vi "UHR-Fleezers Control (host) - 12.7.vi"() -> ()   [LabVIEW 2012] (continued)
                                }
                                frame #6 {
                                n1115 = property on="Rem fb disp offset" class="Bool (strict)"("Val(Sgnl)"=TRUE ("Value (Signaling)")) -> ()  [unwired: 2 in, 2 out]
                                }
                                }
                                }
                                frame True {
                                n1116 = flat-sequence {
                                tunnel: w1651 -> [w1652]
                                frame #0 {
                                n1117 = property on="Trap Delta (MHz)" class="DigNum (strict)"("Val(Sgnl)"=w1652) -> ()  [unwired: 2 in, 2 out]
                                }
                                frame #1 {
                                n1118 = Wait (ms)(milliseconds to wait=u32 500) -> ()  [unwired: 1 out]
                                }
                                frame #2 {
                                n1119 = local read "Shift confocal"() -> (w1658:bool)
                                n1120 = local read "Mean"() -> (w1660:dbl)
                                n1121 = Greater?(x=w1660, y=11.0) -> (0:w1657:bool)
                                n1122 = Not(x=w1657) -> (.not. x?=w1656:bool)
                                n1123 = And(x=w1657, y=w1658) -> (x .and. y?=w1655:bool)
                                n1124 = And(x=w1656, y=w1658) -> (x .and. y?=w1654:bool)
                                n1125 = case shown="True" w1655 {
                                frame False {
                                }
                                frame True {
                                n1126 = local read "Confocal Y 2 (V)"() -> (w1664:dbl)
                                n1127 = local read "Confocal X 2 (V)"() -> (w1663:dbl)
                                n1128 = property on="AO2" class="Slide (strict)"("Val(Sgnl)"=w1663) -> ()  [unwired: 2 in, 2 out]
                                n1129 = property on="AO1" class="Slide (strict)"("Val(Sgnl)"=w1664) -> ()  [unwired: 2 in, 2 out]
                                }
                                }
                                n1130 = case shown="True" w1654 {
                                frame False {
                                }
                                frame True {
                                n1131 = local read "Confocal Y 1 (V)"() -> (w1662:dbl)
                                n1132 = local read "Confocal X 1 (V)"() -> (w1661:dbl)
                                n1133 = property on="AO2" class="Slide (strict)"("Val(Sgnl)"=w1661) -> ()  [unwired: 2 in, 2 out]
                                n1134 = property on="AO1" class="Slide (strict)"("Val(Sgnl)"=w1662) -> ()  [unwired: 2 in, 2 out]
                                }
                                }
                                }
                                }
                                }
                                }
                                }
                                }
                                }
                                }
                                n1135 = local read "Messages"() -> (w1610:string)
                                n1136 = Subtract(x=w1602, y=w1601) -> (x-y=w1608:dbl)
                                "Duration (s)" <- w1608
                                n1137 = Number To Decimal String(number=w1608, width (-)=i16 0) -> (decimal integer string=w1606:string)
                                n1138 = Concatenate Strings(w1606, " s fluorescence event." ("string")) -> (w1604:string)
                                n1139 = call "Update messages.vi"("Message to add"=w1604, "Old message string"=w1610) -> ("New message string"=w1609:string)
                                n1140 = local write "Reset Force"(FALSE ("Reset Force")) -> ()
                                n1141 = local write "Waiting"(TRUE ("Waiting")) -> ()
                                n1142 = local write "Messages"(w1609) -> ()
                                n1143 = local write "Fl. High"(FALSE ("Fl. High")) -> ()
                                n1144 = call <vilib>:"Beep.vi"() -> ()  [unwired: 3 in, 9 out]
                                }
                                }
                                n1145 = node-c288() -> ()  [unwired: 2 out]
                              }
                              n1146 = node-c288(w1578) -> ()  [unwired: 1 out]
                            }
                          }
                        }
                      }
                      n1147 = local read "Trap Delta (MHz)"() -> (w1493:dbl)
                      n1148 = local read "Trap Pos FB SP"() -> (w1488:fxp<+/-,16,1>)
                    }
                  }
                }
                frame #1 {
                  n1149 = local read "Stop All"() -> (w1674:bool)
                  n1150 = local read "Fl. Triggered..."() -> (w1672:bool)
                  n1151 = Not(x=w1672) -> (.not. x?=w1673:bool)
                  n1152 = Or(x=w1673, y=w1674) -> (x .or. y?=w1671:bool)
                }
              }
              n1153 = case shown="True" w1265 {
                frame False {
                }
                frame True {
                  n1154 = local read "Confocal Y 1 (V)"() -> (w1275:dbl)
                  n1155 = local read "Confocal X 1 (V)"() -> (w1274:dbl)
                  n1156 = property on="AO2" class="Slide (strict)"("Val(Sgnl)"=w1274) -> ()  [unwired: 2 in, 2 out]
                  n1157 = property on="AO1" class="Slide (strict)"("Val(Sgnl)"=w1275) -> ()  [unwired: 2 in, 2 out]
                }
              }
              n1158 = case shown="True" w1265 {
                frame False {
                }
                frame True {
                  w1273 = FALSE ("Fl. High")
                  n1159 = local write "Waiting"(w1273) -> ()
                  n1160 = local write "Fl. High"(w1273) -> ()
                }
              }
              n1161 = node-c288() -> ()  [unwired: 2 out]
            }
            n1162 = node-c288(w1263) -> ()  [unwired: 1 out]
          }
        }
      }
      event "Stop All": Value Change {
        n1163 = event-data() -> ()  [unwired: 7 out]
        n1164 = local read "Stop All"() -> (w1679:bool)
      }
    }
    n1165 = node-c288() -> ()  [unwired: 2 out]
  }
  n1166 = timed-loop "Basic control parameters (all FPGA settings, other basic controls)" {
    tunnel: w18 -> [w1688]
    shift-right: [w1687] -> _
    shift-left: errorcluster {"status"=FALSE, "code"=0, "source"=""} ("error out") -> [w1686]
    tunnel: [w1685] -> _
    timing: w128 -> [_]
    timing-out: [_] -> w127
    tunnel: w101 -> [w1684]
    tunnel: w73 -> [w1683]
    tunnel: w72 -> [w1682]
    tunnel: w71 -> [w1681]
    tunnel: w70 -> [w1680]
    stop <- w1685 stop-if-true
    n1167 = node-c288() -> ()  [unwired: 2 out]
    n1168 = event shown="[14] \"DIO count 1 (ticks)\", \"DIO count 2 (ticks)\", \"DIO count 3 (ticks)\", \"Interlace\", \"Number Interlace Sets\", \"Not-Interlacing Set\", \"BD 1 Delay (ticks)\", \"BD 2 Delay (Ticks)\": Value Change" {
      selector: _ -> [_ _ _ _ _ _ _ _ _ _ _ _ _ _ _ _ _ _ _ _ _ _ _ _ _ _ _ _ _ _ _ _ _ _ _ _ _ _ _ _ _ _ _ _ _ _ _ _ _ _ _ _ _ _ _ _ _ _ _ _ _ _ _ _ _ _ _ _ _ _ _ _ _ _]
      dyn-events: _ -> [_ _ _ _ _ _ _ _ _ _ _ _ _ _ _ _ _ _ _ _ _ _ _ _ _ _ _ _ _ _ _ _ _ _ _ _ _ _ _ _ _ _ _ _ _ _ _ _ _ _ _ _ _ _ _ _ _ _ _ _ _ _ _ _ _ _ _ _ _ _ _ _ _ _]
      timeout: _ -> [_ _ _ _ _ _ _ _ _ _ _ _ _ _ _ _ _ _ _ _ _ _ _ _ _ _ _ _ _ _ _ _ _ _ _ _ _ _ _ _ _ _ _ _ _ _ _ _ _ _ _ _ _ _ _ _ _ _ _ _ _ _ _ _ _ _ _ _ _ _ _ _ _ _]
      tunnel: w1688 -> [w1729 _ _ _ w1767 _ w1789 _ _ _ _ w1855 _ _ w1900 w1906 w1913 w1918 w1991 _ w2007 w2032 w2053 w2074 w2094 w2123 w2149 w2152 w2156 w2251 w2256 w2294 _ w2329 w2333 w2344 w2348 w2352 _ w2360 _ _ _ _ _ _ _ _ _ _ _ _ _ _ _ _ _ w2738 _ w2755 _ w2762 w2780 _ w2787 w2795 w2810 w2826 w2832 _ w2841 _ w2860 _]
      tunnel: [w1728 _ _ _ w1757 _ w1788 _ _ w1820 _ w1834 _ _ w1899 w1902 w1912 w1915 w1985 _ w2006 w2031 w2051 w2072 w2092 w2117 w2147 _ w2154 w2249 w2254 w2292 _ w2327 w2331 w2335 w2346 w2350 _ w2358 _ _ _ _ _ _ _ _ _ _ _ _ _ _ _ _ _ w2736 _ _ _ _ w2777 _ _ _ _ _ _ _ _ _ _ _] -> w1687
      tunnel: w1686 -> [w1727 _ _ _ w1766 _ w1787 _ _ w1820 _ w1854 _ _ w1898 w1901 w1911 w1914 w1990 _ w2005 w2030 w2052 w2073 w2093 w2122 w2148 w2151 w2155 w2250 w2255 w2293 _ w2328 w2332 w2343 w2347 w2351 _ w2359 _ _ _ _ _ _ _ _ _ _ _ _ _ _ _ _ _ w2737 _ w2754 _ w2761 w2779 _ w2786 w2794 w2809 w2825 w2831 _ w2840 _ w2859 _]
      tunnel: [_ _ _ _ _ _ _ _ _ w1819 _ _ _ _ _ _ _ _ _ _ _ _ _ _ _ _ _ _ _ _ _ _ _ _ _ _ _ _ _ _ _ _ _ _ _ _ _ _ _ _ _ _ _ _ _ _ _ _ _ _ _ _ _ _ _ _ _ _ _ _ _ _ _ _] -> w1685
      tunnel: [_ _ _ _ _ _ _ "Round T1 X" _ _ _ _ _ _ _ _ _ _ _ _ _ _ _ _ _ _ _ _ _ _ _ _ _ _ _ _ _ _ _ _ _ _ _ _ _ _ _ _ _ _ _ _ _ _ _ _ _ _ _ _ _ _ _ _ _ _ _ _ _ _ _ _ _ _] -> _
      tunnel: [_ _ _ "Adjust Scale\nto Mean" _ _ _ _ _ _ _ _ _ _ _ _ _ _ _ _ _ _ _ _ _ _ _ _ "Test ttrig" _ _ _ _ _ _ _ _ _ _ _ _ _ _ _ _ _ _ "Flush Sample" "Flush Pump 3" "Flush Pump 1" "Clear Volume" _ _ _ _ _ _ _ _ _ _ _ _ _ _ _ _ _ _ _ _ _ _ _] -> _
      tunnel: [_ _ _ _ _ _ _ _ "Round T2 X" _ "Delayed Interlace Start" _ _ _ _ _ _ _ _ _ _ _ _ _ _ _ _ _ _ _ _ _ _ _ _ _ _ _ _ _ _ _ _ _ _ _ _ _ _ _ _ _ _ _ _ _ _ _ _ _ _ _ _ _ _ _ _ _ _ _ _ _ _ _] -> _
      tunnel: w1684 -> [_ _ _ _ _ _ _ _ _ _ _ _ _ _ _ _ _ _ _ _ _ _ _ _ _ _ _ _ _ _ _ _ _ _ _ _ _ _ _ _ _ _ _ w2517 w2524 w2531 w2536 w2545 _ _ w2651 _ _ _ _ _ _ _ _ _ _ _ _ _ _ _ _ _ _ _ _ _ _ _]
      tunnel: w1683 -> [_ _ _ _ _ _ _ _ _ _ _ _ _ _ _ _ _ _ _ _ _ _ _ _ _ _ _ _ _ _ _ _ _ _ _ _ _ _ _ _ _ w2434 _ _ _ _ _ _ w2589 _ _ w2657 _ w2666 _ w2680 _ _ _ _ _ _ _ _ _ _ _ _ _ _ _ _ _ _]
      tunnel: w1682 -> [_ _ _ _ _ _ _ _ _ _ _ _ _ _ _ _ _ _ _ _ _ _ _ _ _ _ _ _ _ _ _ _ _ _ _ _ _ _ _ _ _ _ _ _ _ _ _ _ _ _ _ _ _ _ _ _ _ _ _ _ _ _ _ _ _ _ _ _ _ _ _ _ _ _]
      tunnel: w1681 -> [_ _ _ _ _ _ _ _ _ _ _ _ _ _ _ _ _ _ _ _ _ _ _ _ _ _ _ _ _ _ _ _ _ _ _ _ _ _ _ _ w2371 _ _ _ _ _ _ _ _ w2619 _ _ w2662 _ w2673 _ w2705 _ _ _ _ _ _ _ _ _ _ _ _ _ _ _ _ _]
      tunnel: w1680 -> [_ _ _ _ _ _ _ _ _ _ _ _ _ _ _ _ _ _ _ _ _ _ _ _ _ _ _ _ _ _ _ _ _ _ _ _ _ _ _ _ _ _ _ _ _ _ _ _ _ _ _ _ _ _ _ _ _ _ _ _ _ _ _ _ _ _ _ _ _ _ _ _ _ _]
      event "AI Count (ticks)", "Sets to FIFO (Traps)", "Save ave N", "FPGA Ave.", "# Samples/channel", "N sets to save": Value Change {
        # "So that if 'Save ave N' is updated, the AOD scanning code updates too."
        n1169 = event-data() -> ()  [unwired: 6 out]
        n1170 = local read "AI Count (ticks)"() -> (w1711:u16)
        n1171 = Unbundle By Name("Sets to FIFO (Traps)") -> ("Set 1"=w1694:bool, "Set 2"=w1693:bool, "Set 3"=w1692:bool)
        n1172 = Boolean To (0,1)(Boolean="Sets to FIFO (Traps)") -> (0, 1=w1719:cluster{"Set 1":i16, "Set 2":i16, "Set 3":i16})
        n1173 = xnode "Read/Write Control"("FPGA VI Reference In"=w1729, "error in"=w1727, "ai count"=w1711, "Set 1"=w1694, "Set 2"=w1693, "Set 3"=w1692, "N of AI1 Int Acq Sets"="N Acq Sets (Traps + Fl.)") -> ("error out"=w1728:errorcluster)  [unwired: 1 out]
        n1174 = Cluster To Array(cluster=w1719) -> (array=w1718:i16[])
        n1175 = To Unsigned Long Integer(number=w1718) -> (unsigned 32bit integer=w1700:u32[])
        n1176 = local read "Scan steps (AOD)"() -> (w1720:u64)
        n1177 = Multiply(x=w1711, y="N Acq Sets (Traps + Fl.)") -> (x*y=w1709:u16)
        n1178 = Divide(x=40000000.0, y=w1711) -> (x/y=w1703:dbl)
        "AI rate (Hz)" <- w1703
        "Ave. Rate (Hz)" <- w1703
        n1179 = Add Array Elements(numeric array=w1700) -> (sum=w1712:u32)
        "Trap Sets" <- w1712
        n1180 = Reciprocal(x=w1703) -> (1/x=→"Ave. Period (s)":dbl)
        n1181 = property on="Scan steps (AOD)" class="DigNum (strict)"("Val(Sgnl)"=w1720) -> ()  [unwired: 2 in, 2 out]
        n1182 = Divide(x=w1703, y="N Acq Sets (Traps + Fl.)") -> (x/y=w1724:dbl)
        "Data Rate (Hz)" <- w1724
        n1183 = Reciprocal(x=w1724) -> (1/x=→"Data Period (s)":dbl)
        n1184 = local read "Save ave N"() -> (w1723:dbl)
        n1185 = Divide(x=w1724, y=w1723) -> (x/y=w1722:dbl)
        "Save Data Rate (Hz)" <- w1722
        n1186 = Reciprocal(x=w1722) -> (1/x=→"Save Data Period (s)":dbl)
        n1187 = Multiply(x=w1709, y="# Samples/trap") -> (x*y=w1707:u32)
        "Counts/DMA" <- w1707
        n1188 = property on="Trap Disp. Downsample" class="DigNum (strict)"("Maximum"="# Samples/trap") -> ()  [unwired: 2 in, 2 out]
        n1189 = Multiply(x=w1712, y="# Samples/trap") -> (x*y=w1701:u32)
        "# Samples/channel" <- w1701
        n1190 = Multiply(x=w1701, y=u32 8) -> (x*y=→"Trap AI Elements/DMA read":u32)
        n1191 = local read "APD Int. Count"() -> (w1708:u32)
        n1192 = Multiply(x=w1701, y=u32 3) -> (x*y=→"Trap Pos Elements/DMA read":u32)
        n1193 = Divide(x=w1707, y=w1708) -> (x/y=w1698:dbl)
        "APD Samples/FIFO Acq." <- w1698
        n1194 = Divide(x=w1707, y=40000000.0) -> (x/y=w1705:dbl)
        "DMA Update Period (s)" <- w1705
        n1195 = local read "Number of APDs"() -> (w1691:u8)
        n1196 = Multiply(x=w1691, y=w1698) -> (x*y=→"APD Elements/DMA read":dbl)
        n1197 = property on="APD Disp. Downsample" class="DigNum (strict)"("Maximum"=w1698) -> ()  [unwired: 2 in, 2 out]
        n1198 = local read "N sets to save"() -> (w1717:u32)
        n1199 = Multiply(x=w1705, y=w1717) -> (x*y=→"Total Time (s)":dbl)
        "FPGA Averaging" <- FALSE ("FPGA Averaging")
      }
      event "Remove Offset": Value Change {
        n1200 = event-data() -> ()  [unwired: 7 out]
        n1201 = local write "Remove Offset"(FALSE ("Remove Offset")) -> ()
        n1202 = local read "Bead Mean (nm)"() -> (w1731:dbl)
        n1203 = local read "Offset (nm)"() -> (w1732:dbl)
        n1204 = Add(x=w1731, y=w1732) -> (x+y=w1730:dbl)
        n1205 = local write "Offset (nm)"(w1730) -> ()
        n1206 = disable-structure shown="Disabled" {
          frame Disabled {
            n1207 = local read "Bead Mean (nm)"() -> (w1737:dbl)
            n1208 = Add(y=w1737) -> (x=w1736:dbl, x+y=w1735:dbl)
            n1209 = Subtract(x=w1737, y=w1736) -> (x-y=w1734:dbl)
            n1210 = property on="Bead Separation" class="WFChart (strict)"("YScale.Minimum"=w1734) -> ()  [unwired: 2 in, 2 out]
            n1211 = property on="Bead Separation" class="WFChart (strict)"("YScale.Maximum"=w1735) -> ()  [unwired: 2 in, 2 out]
          }
          frame Enabled {
          }
        }
      }
      event "Detector Type": Value Change {
        n1212 = event-data() -> ()  [unwired: 7 out]
        n1213 = local read "AI labels"() -> (w1738:string[])
        n1214 = property on="High Res. Display" class="Ring (strict)"("Strings []"=w1738) -> ()  [unwired: 2 in, 2 out]
        n1215 = Build Array (concatenate)(w1738, "none") -> (w1739:string[])
        n1216 = property on="FFT 1 Choice 1" class="Ring (strict)"("Strings []"=w1739) -> ()  [unwired: 2 in, 2 out]
        n1217 = property on="FFT 1 Choice 2" class="Ring (strict)"("Strings []"=w1739) -> ()  [unwired: 2 in, 2 out]
        n1218 = property on="FFT 2 Choice 1" class="Ring (strict)"("Strings []"=w1739) -> ()  [unwired: 2 in, 2 out]
        n1219 = property on="FFT 2 Choice 2" class="Ring (strict)"("Strings []"=w1739) -> ()  [unwired: 2 in, 2 out]
        n1220 = Bundle("APD 1", "APD 2") -> (w1742:cluster{string, string})  [unwired: 1 out]
        n1221 = Cluster To Array(cluster=w1742) -> (array=w1740:string[])
        n1222 = Build Array (concatenate)(w1740, w1739) -> (w1744:string[])
        n1223 = Array Size(array=w1744) -> (size(s)=w1745:i32)
        n1224 = property on="Signals to Plot" class="LstBox (strict)"("Item Names"=w1744) -> ()  [unwired: 2 in, 2 out]
        n1225 = property on="Signals to Plot" class="LstBox (strict)"("Number of Rows"=w1745) -> ()  [unwired: 2 in, 2 out]
        n1226 = property on="All Signals" class="WFChart (strict)"("LegNumRows"=w1745) -> ()  [unwired: 2 in, 2 out]
      }
      event "Adjust Scale\nto Mean": Value Change {
        n1227 = event-data() -> ()  [unwired: 7 out]
        n1228 = local read "APD 1 Rate (Hz)"() -> (w1754:dbl)
        n1229 = Multiply(x=1000.0, y="Above (kHz)") -> (x*y=w1752:dbl)
        n1230 = Multiply(x=1000.0, y="Below (kHz)") -> (x*y=w1750:dbl)
        n1231 = Add(x=w1752, y=w1754) -> (x+y=w1747:dbl)
        n1232 = Subtract(x=w1754, y=w1750) -> (x-y=w1748:dbl)
        n1233 = property on="APD Chart" class="WFChart (strict)"("YScale.Minimum"=w1748) -> ()  [unwired: 2 in, 2 out]
        n1234 = property on="APD Chart" class="WFChart (strict)"("YScale.Maximum"=w1747) -> ()  [unwired: 2 in, 2 out]
      }
      event "Phase adj. (AI1)", "+ phase (AI1)", "- phase (AI1)": Value Change {
        n1235 = event-data() -> ()  [unwired: 7 out]
        n1236 = Negate(x="Phase adj. (AI1)") -> (-x=w1764:i16)
        n1237 = Select(t=w1764, s="- phase (AI1)", f="Phase adj. (AI1)") -> (s? t:f=w1763:i16)
        n1238 = xnode "Read/Write Control"("FPGA VI Reference In"=w1767, "error in"=w1766, "Phase count adjustment"=w1763) -> ("FPGA VI Reference Out"=w1762:T20, "error out"=w1761:errorcluster)  [unwired: 1 in]
        n1239 = Or(x="- phase (AI1)", y="+ phase (AI1)") -> (x .or. y?=w1758:bool)
        n1240 = xnode "Read/Write Control"("FPGA VI Reference In"=w1762, "error in"=w1761, "+ phase"=w1758) -> ("error out"=w1757:errorcluster)  [unwired: 1 in, 1 out]
      }
      event "Signals to Plot": Double Click {
        w1770 = u32 9868950 ("Color Box")
        n1241 = event-data() -> ("Row"=w1772:i32)  [unwired: 9 out]
        n1242 = property on="All Signals" class="WFChart (strict)"("Active Plot"=w1772) -> (error out=w1783:errorcluster)  [unwired: 2 in, 1 out]
        n1243 = property on="All Signals" class="WFChart (strict)" props=["Plot", "Visible?", "Plot", "Plot Color"](error in=w1783) -> (error out=w1782:errorcluster, "Plot.Visible?"=w1781:bool)  [unwired: 1 in, 2 out]
        n1244 = Select(t=FALSE ("Plot.Visible"), s=w1781, f=TRUE ("Plot.Visible")) -> (s? t:f=w1776:bool)
        n1245 = property on="All Signals" class="WFChart (strict)"(error in=w1782, "Plot.Visible?"=w1776) -> (error out=w1778:errorcluster)  [unwired: 1 in, 1 out]
        n1246 = property on="All Signals" class="WFChart (strict)"(error in=w1778) -> (error out=w1773:errorcluster, "Plot.Plot Color"=w1777:u32)  [unwired: 1 in, 1 out]
        n1247 = property on="Signals to Plot" class="LstBox (strict)"(error in=w1773, "Active Row"=w1772) -> (error out=w1771:errorcluster)  [unwired: 1 in, 1 out]
        n1248 = Select(t=w1777, s=w1776, f=u32 0) -> (s? t:f=w1774:u32)
        n1249 = property on="Signals to Plot" class="LstBox (strict)"(error in=w1771, "CellFontColor"=w1774, "SelColor"=w1770, "CellBG"=w1770, "CellFontSize"=u32 20 ("Active Row:Cell Font:Size"), "CellFontBold"=TRUE ("Active Row:Cell Font:Bold")) -> ()  [unwired: 1 in, 2 out]
      }
      event "BD 1 Frequency 1 (MHz)", "BD 1 Frequency 2 (MHz)", "BD 1 Frequency 3 (MHz)", "BD 2 Frequency 1 (MHz)", "BD 2 Frequency 2 (MHz)", "BD 2 Frequency 3 (MHz)", "Trap Delta (MHz)": Value Change {
        n1250 = event-data() -> ("CtlRef"=w1786:refnum<vi>)  [unwired: 6 out]
        n1251 = control-ref of="Trap Delta (MHz)"() -> (w1785:refnum<vi>)
        n1252 = Equal?(x=w1785, y=w1786) -> (x = y?=w1784:bool)
        n1253 = case shown="False" "Oscillate Set 1" {
          tunnel: w1789 -> [w1809 _]
          tunnel: [w1808 w1812] -> w1788
          tunnel: w1787 -> [w1807 w1812]
          tunnel: w1784 -> [w1792 _]
          frame False {
            n1254 = local read "BD 1 Frequency 2 (MHz)"() -> (w1796:dbl)
            n1255 = local read "BD 1 Frequency 1 (MHz)"() -> (w1794:dbl)
            n1256 = Subtract(x=w1796, y="Trap Delta (MHz)") -> (x-y=w1793:dbl)
            n1257 = Select(t=w1793, s=w1792, f=w1794) -> (s? t:f=w1791:dbl)
            n1258 = local read "Y RF Frequency Limits (MHz)"() -> (w1797:T16)
            n1259 = local read "X RF Frequency Limits (MHz)"() -> (w1798:T16)
            n1260 = local read "BD 1 Frequency 3 (MHz)"() -> (w1810:dbl)
            n1261 = local write "BD 1 Frequency 1 (MHz)"(w1791) -> ()
            n1262 = local read "BD 2 Frequency 1 (MHz)"() -> (w1801:dbl)
            n1263 = local read "BD 2 Frequency 2 (MHz)"() -> (w1800:dbl)
            n1264 = local read "BD 2 Frequency 3 (MHz)"() -> (w1811:dbl)
            n1265 = call "set RF board frequency - interlace.vi"("Board 2 Frequency Limits"=w1797, "Board 1 Frequency Limits"=w1798, "error in"=w1807, "FPGA VI Reference In"=w1809, "Board 2 Frequency 3 (MHz)"=w1811, "Board 1 Frequency 3 (MHz)"=w1810, "Board 2 Frequency 2 (MHz)"=w1800, "Board 2 Frequency 1 (MHz)"=w1801, "Board 1 Frequency 2 (MHz)"=w1796, "Board 1 Frequency 1  (MHz)"=w1791) -> ("error out"=w1808:errorcluster)  [unwired: 1 out]
            n1266 = Subtract(x=w1801, y=w1800) -> (x-y=w1805:dbl)
            n1267 = Subtract(x=w1791, y=w1796) -> (x-y=w1806:dbl)
            n1268 = Square(x=w1805) -> (x^2=w1803:dbl)
            n1269 = Square(x=w1806) -> (x^2=w1804:dbl)
            n1270 = Add(x=w1804, y=w1803) -> (x+y=w1802:dbl)
            n1271 = Square Root(x=w1802) -> (sqrt(x)=w1799:dbl)
            n1272 = local write "Trap Delta (MHz)"(w1799) -> ()
            n1273 = property on="Initial delta (MHz)" class="DigNum (strict)"("Val(Sgnl)"=w1799) -> ()  [unwired: 2 in, 2 out]
          }
          frame True {
          }
        }
      }
      event "Round T1 X": Value Change {
        n1274 = event-data() -> ()  [unwired: 7 out]
        n1275 = local read "BD 1 Frequency 1 (MHz)"() -> (w1815:dbl)
        n1276 = Round To Nearest(number=w1815) -> (nearest integer value=w1814:dbl)
        n1277 = property on="BD 1 Frequency 1 (MHz)" class="DigNum (strict)"("Val(Sgnl)"=w1814) -> ()  [unwired: 2 in, 2 out]
      }
      event "Round T2 X": Value Change {
        n1278 = event-data() -> ()  [unwired: 7 out]
        n1279 = local read "BD 1 Frequency 2 (MHz)"() -> (w1817:dbl)
        n1280 = Round To Nearest(number=w1817) -> (nearest integer value=w1816:dbl)
        n1281 = property on="BD 1 Frequency 2 (MHz)" class="DigNum (strict)"("Val(Sgnl)"=w1816) -> ()  [unwired: 2 in, 2 out]
      }
      event "Stop All": Value Change {
        n1282 = event-data() -> ()  [unwired: 7 out]
        n1283 = local read "Stop All"() -> (w1819:bool)
      }
      event "Delayed Interlace Start": Value Change {
        n1284 = event-data() -> ()  [unwired: 7 out]
        n1285 = flat-sequence {
          frame #0 {
            n1286 = Multiply(x="Delay to Interlace (s)", y=1000.0) -> (x*y=w1822:dbl)
            n1287 = Wait (ms)(milliseconds to wait=w1822) -> ()  [unwired: 1 out]
          }
          frame #1 {
            n1288 = property on="Laser interlacing mode" class="RadioBtnsControl (strict)"("Val(Sgnl)"=enum32{"Laser ON", "Laser OFF", "Interlace"}."Interlace" ("Value (Signaling)")) -> ()  [unwired: 2 in, 2 out]
          }
        }
      }
      event "BD 1 Amplitude 1 (%)", "BD 1 Amplitude 2 (%)", "BD 1 Amplitude 3 (%)", "BD 2 Amplitude 1 (%)", "BD 2 Amplitude 2 (%)", "BD 2 Amplitude 3 (%)", "Trap 1 ON", "Trap 2 ON", "Trap 3 ON", "Feedback On/Off", "All FB On/Off": Value Change {
        w1846 = i16 1 ("f")
        n1289 = event-data() -> ()  [unwired: 7 out]
        n1290 = local write "Trap 1 (ON/OFF)"("Trap 1 ON") -> ()
        n1291 = local write "Trap 2 (ON/OFF)"("Trap 2 ON") -> ()
        n1292 = Boolean To (0,1)(Boolean="Trap 3 ON") -> (0, 1=w1847:i16)
        n1293 = Boolean To (0,1)(Boolean="Trap 1 ON") -> (0, 1=w1848:i16)
        n1294 = Boolean To (0,1)(Boolean="Trap 2 ON") -> (0, 1=w1849:i16)
        n1295 = Select(t=w1849, s="Trap ON/OFF X or Y Amp?", f=w1846) -> (s? t:f=w1844:i16)
        n1296 = Select(t=w1848, s="Trap ON/OFF X or Y Amp?", f=w1846) -> (s? t:f=w1845:i16)
        n1297 = Select(t=w1847, s="Trap ON/OFF X or Y Amp?", f=w1846) -> (s? t:f=w1843:i16)
        n1298 = Select(t=w1846, s="Trap ON/OFF X or Y Amp?", f=w1849) -> (s? t:f=w1841:i16)
        n1299 = Select(t=w1846, s="Trap ON/OFF X or Y Amp?", f=w1848) -> (s? t:f=w1842:i16)
        n1300 = Select(t=w1846, s="Trap ON/OFF X or Y Amp?", f=w1847) -> (s? t:f=w1840:i16)
        n1301 = And(x="All FB On/Off", y="Feedback On/Off") -> (x .and. y?=w1838:cluster{"Set 1":bool, "Set 2":bool})
        n1302 = local read "BD 1 Amplitude 1 (%)"() -> (w1858:dbl)
        n1303 = local read "BD 1 Amplitude 2 (%)"() -> (w1857:dbl)
        n1304 = local read "BD 1 Amplitude 3 (%)"() -> (w1856:dbl)
        n1305 = Unbundle By Name(w1838) -> ("Set 1"=w1833:bool, "Set 2"=w1830:bool)
        n1306 = local read "Y RF Amplitude Limits (%)"() -> (w1826:T16)
        n1307 = local read "X RF Amplitude Limits (%)"() -> (w1827:T16)
        n1308 = local read "BD 2 Amplitude 1 (%)"() -> (w1859:dbl)
        n1309 = local read "BD 2 Amplitude 2 (%)"() -> (w1860:dbl)
        n1310 = local read "BD 2 Amplitude 3 (%)"() -> (w1861:dbl)
        n1311 = And(x="Trap 2 ON", y=w1830) -> (x .and. y?=w1828:bool)
        n1312 = And(x="Trap 1 ON", y=w1833) -> (x .and. y?=w1831:bool)
        n1313 = Multiply(x=w1845, y=w1858) -> (x*y=w1853:dbl)
        n1314 = Multiply(x=w1857, y=w1844) -> (x*y=w1851:dbl)
        n1315 = Multiply(x=w1856, y=w1843) -> (x*y=w1852:dbl)
        n1316 = Multiply(x=w1859, y=w1842) -> (x*y=w1862:dbl)
        n1317 = Multiply(x=w1860, y=w1841) -> (x*y=w1863:dbl)
        n1318 = Multiply(x=w1861, y=w1840) -> (x*y=w1864:dbl)
        n1319 = call "set RF board amplitude - interlace.vi"("Board 2 Amplitude Limits"=w1826, "Board 1 Amplitude Limits"=w1827, "error in"=w1854, "FPGA VI Reference In"=w1855, "Board 2 Amplitude 3 (%)"=w1864, "Board 1 Amplitude 3 (%)"=w1852, "Board 2 Amplitude 2 (%)"=w1863, "Board 2 Amplitude 1 (%)"=w1862, "Board 1 Amplitude 2 (%)"=w1851, "Board 1 Amplitude 1 (%)"=w1853) -> ("error out"=w1835:errorcluster, "FPGA VI Reference Out"=w1836:T20)
        n1320 = xnode "Read/Write Control"("FPGA VI Reference In"=w1836, "error in"=w1835, "FB On/Off Set 1"=w1831, "FB On/Off Set 2"=w1828) -> ("error out"=w1834:errorcluster)  [unwired: 1 out]
      }
      event "Load parameters": Value Change {
        n1321 = event-data() -> ()  [unwired: 7 out]
        n1322 = property on="Saved AOD Raster Scan Parameter Sets" class="Arr (strict)"() -> ("Index Values"=w1875:u32[])  [unwired: 2 in, 2 out]
        n1323 = Index Array(array=w1875, index=0) -> (element=w1872:u32)
        n1324 = local write "Load parameters"(FALSE ("Load parameters")) -> ()
        n1325 = Index Array(array="Saved AOD Raster Scan Parameter Sets", index=w1872) -> (element=w1871:T30)
        n1326 = Unbundle By Name(w1871) -> ("Scan Range AOD (nm) 2"=w1870:dbl, "Step Size AOD (nm) 2"=w1869:dbl, "Scan Speed AOD (nm/s) 2"=w1868:dbl, "Number of scans (AOD) 2"=w1867:u16)
        n1327 = flat-sequence {
          tunnel: w1870 -> [w1878]
          tunnel: w1869 -> [w1877]
          tunnel: w1868 -> [w1876]
          tunnel: w1867 -> [w1879]
          frame #0 {
            n1328 = local write "Scan Speed (nm/s)"(w1876) -> ()
            n1329 = local write "Scan Range (nm)"(w1878) -> ()
            n1330 = local write "Step Size (nm)"(w1877) -> ()
          }
          frame #1 {
            n1331 = property on="Number of F/B Scans (AOD)" class="DigNum (strict)"("Val(Sgnl)"=w1879) -> ()  [unwired: 2 in, 2 out]
          }
        }
      }
      event "Trap 1 (ON/OFF)", "Trap 2 (ON/OFF)": Value Change {
        n1332 = event-data() -> ()  [unwired: 7 out]
        n1333 = property on="Trap 2 ON" class="Bool (strict)"("Val(Sgnl)"="Trap 2 (ON/OFF)") -> ()  [unwired: 2 in, 2 out]
        n1334 = property on="Trap 1 ON" class="Bool (strict)"("Val(Sgnl)"="Trap 1 (ON/OFF)") -> ()  [unwired: 2 in, 2 out]
      }
      event "DIO count 1 (ticks)", "DIO count 2 (ticks)", "DIO count 3 (ticks)", "Interlace", "Number Interlace Sets", "Not-Interlacing Set", "BD 1 Delay (ticks)", "BD 2 Delay (Ticks)": Value Change {
        n1335 = event-data() -> ()  [unwired: 7 out]
        n1336 = local read "DIO count 3 (ticks)"() -> (w1894:u16)
        n1337 = local read "DIO count 1 (ticks)"() -> (w1896:u16)
        n1338 = local read "DIO count 2 (ticks)"() -> (w1895:u16)
        n1339 = To Unsigned Byte Integer(number="Not-Interlacing Set") -> (unsigned 8bit integer=w1885:u8)
        n1340 = Add(x=w1885, y=u8 1) -> (x+y=w1889:u8)
        n1341 = xnode "Read/Write Control"("FPGA VI Reference In"=w1900, "error in"=w1898, "DIO count 1 (ticks)"=w1896, "DIO count 2 (ticks)"=w1895, "DIO count 3 (ticks)"=w1894, "Interlace ON/OFF"="Interlace", "Number Interlace Cycles"="Number Interlace Sets", "Interlace Off Parameters"=w1889, "BD 1 Delay (ticks)"="BD 1 Delay (ticks)", "BD 2 Delay (Ticks)"="BD 2 Delay (Ticks)") -> ("error out"=w1899:errorcluster)  [unwired: 1 out]
        n1342 = Build Array(w1896, w1895, w1894) -> (w1887:u16[])
        n1343 = Split 1D Array(array=w1887, index="Number Interlace Sets") -> (first subarray=w1897:u16[])  [unwired: 1 out]
        n1344 = Index Array(array=w1887, index=w1885) -> (element=w1886:u16)
        n1345 = Add Array Elements(numeric array=w1897) -> (sum=w1891:u16)
        n1346 = Select(t=w1891, s="Interlace", f=w1886) -> (s? t:f=→"Total Counts (ticks)":u16)
      }
      event "Reset Feedback": Value Change {
        n1347 = event-data() -> ()  [unwired: 7 out]
        n1348 = Unbundle By Name("Reset Feedback") -> ("Set 1"=w1904:bool, "Set 2"=w1903:bool)
        n1349 = xnode "Read/Write Control"("FPGA VI Reference In"=w1906, "error in"=w1901, "FB Reset Set 1"=w1904, "FB Reset Set 2"=w1903) -> ("error out"=w1902:errorcluster)  [unwired: 1 out]
      }
      event "Trap Intensity PID Gains": Value Change {
        n1350 = event-data() -> ()  [unwired: 7 out]
        n1351 = Unbundle By Name("Trap Intensity PID Gains") -> ("proportional gain (Kc)"=w1909:i16, "integral gain (Kc*Ts/Ti)"=w1908:i16, "derivative gain (Kc*Td/Ts)"=w1907:i16)
        n1352 = xnode "Read/Write Control"("FPGA VI Reference In"=w1913, "error in"=w1911, "P1"=w1909, "I1"=w1908, "D1"=w1907) -> ("error out"=w1912:errorcluster)  [unwired: 1 out]
      }
      event "AI2 to Setpoint", "Setpoints (V)": Value Change {
        n1353 = event-data() -> ()  [unwired: 7 out]
        n1354 = xnode "Read/Write Control"("FPGA VI Reference In"=w1918, "error in"=w1914) -> ("FPGA VI Reference Out"=w1917:T20, "error out"=w1916:errorcluster, "AI2 Y Sum Set 1"=w1925:i16, "AI2 Y Sum Set 2"=w1924:i16)
        n1355 = Cluster To Array(cluster="AI2 to Setpoint") -> (array=w1928:bool[])
        n1356 = local read "AI2 (V)"() -> (w1926:cluster{"Set 1":dbl, "Set 2":dbl})
        n1357 = Or Array Elements(Boolean array=w1928) -> (logical OR=w1929:bool)
        n1358 = Bundle By Name(cluster=w1926, "Set 1"=w1925, "Set 2"=w1924) -> (w1923:cluster{"Set 1":dbl, "Set 2":dbl})
        n1359 = Divide(x=w1923, y=3276.7) -> (x/y=w1922:cluster{"Set 1":dbl, "Set 2":dbl})
        "AI2 (V)" <- w1922
        n1360 = case shown="True" w1929 {
          tunnel: [w1932 w1949] -> w1921
          tunnel: "AI2 to Setpoint" -> [_ w1945]
          tunnel: "Setpoints (V)" -> [w1933 w1948]
          tunnel: w1922 -> [_ w1942]
          frame False {
            n1361 = Multiply(x=3276.7, y=w1933) -> (x*y=w1934:cluster{"Set 1":dbl, "Set 2":dbl})
            n1362 = To Word Integer(number=w1934) -> (16bit integer=w1932:cluster{"Set 1":i16, "Set 2":i16})
          }
          frame True {
            n1363 = Unbundle By Name(w1942) -> ("Set 1"=w1941:dbl, "Set 2"=w1940:dbl)
            n1364 = Unbundle By Name(w1948) -> ("Set 1"=w1947:dbl, "Set 2"=w1946:dbl)
            n1365 = Unbundle By Name(w1945) -> ("Set 1"=w1944:bool, "Set 2"=w1943:bool)
            n1366 = Select(t=w1941, s=w1944, f=w1947) -> (s? t:f=w1939:dbl)
            n1367 = Select(t=w1940, s=w1943, f=w1946) -> (s? t:f=w1938:dbl)
            n1368 = Bundle By Name(cluster=w1948, "Set 1"=w1939, "Set 2"=w1938) -> (w1936:cluster{"Set 1":dbl, "Set 2":dbl})
            n1369 = local write "Setpoints (V)"(w1936) -> ()
            n1370 = Multiply(x=3276.7, y=w1936) -> (x*y=w1937:cluster{"Set 1":dbl, "Set 2":dbl})
            n1371 = To Word Integer(number=w1937) -> (16bit integer=w1949:cluster{"Set 1":i16, "Set 2":i16})
          }
        }
        n1372 = Unbundle By Name(w1921) -> ("Set 1"=w1920:i16, "Set 2"=w1919:i16)
        n1373 = xnode "Read/Write Control"("FPGA VI Reference In"=w1917, "error in"=w1916, "FB Setpoint Set 1"=w1920, "FB Setpoint Set 2"=w1919) -> ("error out"=w1915:errorcluster)  [unwired: 1 out]
      }
      event "+ phase (GI)", "- phase (GI)", "+ phase (GI) 2", "- phase (GI) 2", "+ phase (RI)", "- phase (RI)", "+ phase (Green FB)", "- phase (Green FB)": Value Change {
        n1374 = event-data() -> ()  [unwired: 7 out]
        n1375 = Or(x="+ phase (GI)", y="- phase (GI)") -> (x .or. y?=w1984:bool)
        n1376 = Negate(x="Phase adj. (GI)") -> (-x=w1989:i16)
        n1377 = Select(t=w1989, s="+ phase (GI)", f="Phase adj. (GI)") -> (s? t:f=w1988:i16)
        n1378 = Or(x="+ phase (GI) 2", y="- phase (GI) 2") -> (x .or. y?=w1975:bool)
        n1379 = Negate(x="Phase adj. (GI) 2") -> (-x=w1980:i16)
        n1380 = Select(t=w1980, s="+ phase (GI) 2", f="Phase adj. (GI) 2") -> (s? t:f=w1976:i16)
        n1381 = Negate(x="Phase adj. (RI)") -> (-x=w1974:i16)
        n1382 = Or(x="+ phase (RI)", y="- phase (RI)") -> (x .or. y?=w1970:bool)
        n1383 = Select(t=w1974, s="+ phase (RI)", f="Phase adj. (RI)") -> (s? t:f=w1969:i16)
        n1384 = Or(x="+ phase (Green FB)", y="- phase (Green FB)") -> (x .or. y?=w1963:bool)
        n1385 = Negate(x="Phase adj. (Green FB)") -> (-x=w1968:i16)
        n1386 = Select(t=w1968, s="+ phase (Green FB)", f="Phase adj. (Green FB)") -> (s? t:f=w1964:i16)
        n1387 = Negate(x="Phase adj. (BI AO)") -> (-x=w1962:i16)
        n1388 = Or(x="+ phase (BI AO)", y="- phase (BI AO)") -> (x .or. y?=w1952:bool)
        n1389 = Select(t=w1962, s="+ phase (BI AO)", f="Phase adj. (BI AO)") -> (s? t:f=w1954:i16)
        n1390 = Negate(x="Phase adj. (BI DO)") -> (-x=w1958:i16)
        n1391 = Or(x="+ phase (BI DO)", y="- phase (BI DO)") -> (x .or. y?=w1951:bool)
        n1392 = Select(t=w1958, s="+ phase (BI DO)", f="Phase adj. (BI DO)") -> (s? t:f=w1953:i16)
        n1393 = xnode "Read/Write Control"("FPGA VI Reference In"=w1991, "error in"=w1990, "Phase count adjustment (GI)"=w1988, "Phase count adjustment (GI) 2"=w1976, "Phase count adjustment (RI)"=w1969, "Phase count adjustment (Green FB)"=w1964, "Phase count adjustment (BI AO)"=w1954, "Phase count adjustment (BI D)"=w1953) -> ("FPGA VI Reference Out"=w1986:T20, "error out"=w1987:errorcluster)
        n1394 = xnode "Read/Write Control"("FPGA VI Reference In"=w1986, "error in"=w1987, "+ phase (GI)"=w1984, "+ phase (GI) 2"=w1975, "+ phase (RI)"=w1970, "+ phase (Green FB)"=w1963, "+ phase (BI AO)"=w1952, "+ phase (BI D)"=w1951) -> ("error out"=w1985:errorcluster)  [unwired: 1 out]
      }
      event "Green Laser ON/OFF", "Red Laser ON/OFF", "Blue Laser ON/OFF": Value Change {
        # "This loop shouldn't be initialized.  The main 'laser ON' settings should dominate and set the others."
        n1395 = event-data() -> ()  [unwired: 7 out]
        n1396 = property on="Red Laser ON" class="Bool (strict)"("Val(Sgnl)"="Red Laser ON/OFF") -> ()  [unwired: 2 in, 2 out]
        n1397 = property on="Blue Laser ON" class="Bool (strict)"("Val(Sgnl)"="Blue Laser ON/OFF") -> ()  [unwired: 2 in, 2 out]
        n1398 = property on="Green Laser ON" class="Bool (strict)"("Val(Sgnl)"="Green Laser ON/OFF") -> ()  [unwired: 2 in, 2 out]
      }
      event "Laser interlacing mode", "Green Laser ON", "Red Laser ON", "Blue Laser ON": Value Change {
        n1399 = event-data() -> ()  [unwired: 7 out]
        n1400 = local write "Green Laser ON/OFF"("Green Laser ON") -> ()
        n1401 = local write "Blue Laser ON/OFF"("Blue Laser ON") -> ()
        n1402 = local write "Red Laser ON/OFF"("Red Laser ON") -> ()
        n1403 = case shown="True" "Green Laser ON" {
          tunnel: "Laser interlacing mode" -> [_ w2028]
          tunnel: [enum32{"Laser ON", "Laser OFF", "Interlace"}."Laser OFF" ("Green laser mode") w2028] -> w2004
          tunnel: [FALSE w2024] -> w2003
          frame False {
          }
          frame True {
            n1404 = local read "Green FB On/Off"() -> (w2025:bool)
            n1405 = Equal?(x=w2028, y=enum32{"Laser ON", "Laser OFF", "Interlace"}."Interlace") -> (x = y?=w2026:bool)
            n1406 = And(x=w2026, y=w2025) -> (x .and. y?=w2024:bool)
          }
        }
        n1407 = case shown="True" "Red Laser ON" {
          tunnel: "Laser interlacing mode" -> [_ w2021]
          tunnel: [enum32{"Laser ON", "Laser OFF", "Interlace"}."Laser OFF" ("Green laser mode") w2021] -> w2000
          tunnel: [FALSE w2017] -> w1999
          frame False {
          }
          frame True {
            n1408 = local read "Red FB On/Off"() -> (w2018:bool)
            n1409 = Equal?(x=w2021, y=enum32{"Laser ON", "Laser OFF", "Interlace"}."Interlace") -> (x = y?=w2019:bool)
            n1410 = And(x=w2019, y=w2018) -> (x .and. y?=w2017:bool)
          }
        }
        n1411 = case shown="True" "Blue Laser ON" {
          tunnel: "Laser interlacing mode" -> [_ w2012]
          tunnel: [enum32{"Laser ON", "Laser OFF", "Interlace"}."Laser OFF" ("Green laser mode") w2012] -> w1996
          tunnel: [FALSE w2010] -> w1995
          frame False {
          }
          frame True {
            n1412 = local read "Blue FB On/Off"() -> (w2011:bool)
            n1413 = Equal?(x=w2012, y=enum32{"Laser ON", "Laser OFF", "Interlace"}."Interlace") -> (x = y?=w2013:bool)
            n1414 = And(x=w2013, y=w2011) -> (x .and. y?=w2010:bool)
          }
        }
        n1415 = xnode "Read/Write Control"("FPGA VI Reference In"=w2007, "error in"=w2005, "Operating Mode"=w2004, "Operating Mode 2"=w2004, "Green FB On/Off"=w2003, "Red Laser Operating Mode"=w2000, "RI Operating Mode 2"=w2000, "Red FB On/Off"=w1999, "BI Operating Mode (AO)"=w1996, "Blue Laser Operating Mode (D)"=w1996, "Blue FB On/Off"=w1995) -> ("error out"=w2006:errorcluster)  [unwired: 1 out]
      }
      event "Invert laser interlacing": Value Change {
        n1416 = event-data() -> ()  [unwired: 7 out]
        n1417 = xnode "Read/Write Control"("FPGA VI Reference In"=w2032, "error in"=w2030, "Invert GI"="Invert laser interlacing", "Invert GI 2"="Invert laser interlacing", "Invert RI"="Invert laser interlacing", "Invert RI 2"="Invert laser interlacing", "Invert BI (AO)"="Invert laser interlacing", "Invert BI (D)"="Invert laser interlacing") -> ("error out"=w2031:errorcluster)  [unwired: 1 out]
      }
      event "Green FB Setpoint (mV)", "Green FB Gains", "Green FB On/Off", "Green Intensity % (FB OFF)", "Green int current ON count adj": Value Change {
        n1418 = event-data() -> ()  [unwired: 7 out]
        n1419 = local read "Green FB Setpoint (mV)"() -> (w2043:dbl)
        n1420 = Multiply(x=w2043, y=3.2767) -> (x*y=w2042:dbl)
        n1421 = local read "Green Intensity % (FB OFF)"() -> (w2046:dbl)
        n1422 = Multiply(x=w2046, y=655.35) -> (x*y=w2047:dbl)
        n1423 = To Unsigned Word Integer(number=w2047) -> (unsigned 16bit integer=w2045:u16)
        n1424 = local read "Green int current ON count adj"() -> (w2049:u32)
        n1425 = local read "Laser interlacing mode"() -> (w2039:enum32{"Laser ON", "Laser OFF", "Interlace"})
        n1426 = local read "Green FB Gains"() -> (w2036:T9)
        n1427 = local read "Green Laser ON"() -> (w2040:bool)
        n1428 = local read "Green FB On/Off"() -> (w2050:bool)
        n1429 = Equal?(x=w2039, y=enum32{"Laser ON", "Laser OFF", "Interlace"}."Interlace") -> (x = y?=w2037:bool)
        n1430 = Unbundle By Name(w2036) -> ("proportional gain (Kc)"=w2035:i16, "integral gain (Kc*Ts/Ti)"=w2034:i16, "derivative gain (Kc*Td/Ts)"=w2033:i16)
        n1431 = Compound Arithmetic op=AND(w2037, w2050, w2040) -> (w2041:bool)
        n1432 = xnode "Read/Write Control"("FPGA VI Reference In"=w2053, "error in"=w2052, "Green FB Setpoint"=w2042, "Green FB On/Off"=w2041, "Current Out"=w2045, "Green int current ON count adj"=w2049, "P3"=w2035, "I3"=w2034, "D3"=w2033) -> ("error out"=w2051:errorcluster)  [unwired: 1 out]
      }
      event "Blue FB Setpoint (mV)", "Blue FB Gains", "Blue FB On/Off", "Blue Intensity % (FB OFF)", "Blue int AO ON count adjust": Value Change {
        # "16 bit analog out"
        n1433 = event-data() -> ()  [unwired: 7 out]
        n1434 = Multiply(x="Blue FB Setpoint (mV)", y=3.2767) -> (x*y=w2067:dbl)
        n1435 = Multiply(x="Blue Intensity % (FB OFF)", y=655.35) -> (x*y=w2070:dbl)
        n1436 = To Unsigned Word Integer(number=w2070) -> (unsigned 16bit integer=w2069:u16)
        n1437 = local read "Laser interlacing mode"() -> (w2065:enum32{"Laser ON", "Laser OFF", "Interlace"})
        n1438 = Unbundle By Name("Blue FB Gains") -> ("proportional gain (Kc)"=w2062:i16, "integral gain (Kc*Ts/Ti)"=w2061:i16, "derivative gain (Kc*Td/Ts)"=w2060:i16)
        n1439 = local read "Blue Laser ON"() -> (w2054:bool)
        n1440 = Equal?(x=w2065, y=enum32{"Laser ON", "Laser OFF", "Interlace"}."Interlace") -> (x = y?=w2063:bool)
        n1441 = Compound Arithmetic op=AND(w2063, "Blue FB On/Off", w2054) -> (w2066:bool)
        n1442 = xnode "Read/Write Control"("FPGA VI Reference In"=w2074, "error in"=w2073, "Blue FB Setpoint"=w2067, "Blue FB On/Off"=w2066, "BI Current Out"=w2069, "Blue current ON count adj (AO)"="Blue int AO ON count adjust", "P5"=w2062, "I5"=w2061, "D5"=w2060) -> ("error out"=w2072:errorcluster)  [unwired: 1 out]
      }
      event "Red FB Setpoint (mV)", "Red FB Gains", "Red FB On/Off", "Red Intensity % (FB OFF)": Value Change {
        n1443 = event-data() -> ()  [unwired: 7 out]
        n1444 = local read "Red FB Setpoint (mV)"() -> (w2086:dbl)
        n1445 = Multiply(x=w2086, y=3.2767) -> (x*y=w2085:dbl)
        n1446 = local read "Red Intensity % (FB OFF)"() -> (w2075:dbl)
        n1447 = Multiply(x=w2075, y=655.35) -> (x*y=w2089:dbl)
        n1448 = To Unsigned Word Integer(number=w2089) -> (unsigned 16bit integer=w2088:u16)
        n1449 = local read "Laser interlacing mode"() -> (w2082:enum32{"Laser ON", "Laser OFF", "Interlace"})
        n1450 = local read "Red FB Gains"() -> (w2079:T9)
        n1451 = local read "Red Laser ON"() -> (w2083:bool)
        n1452 = local read "Red FB On/Off"() -> (w2091:bool)
        n1453 = Equal?(x=w2082, y=enum32{"Laser ON", "Laser OFF", "Interlace"}."Interlace") -> (x = y?=w2080:bool)
        n1454 = Unbundle By Name(w2079) -> ("proportional gain (Kc)"=w2078:i16, "integral gain (Kc*Ts/Ti)"=w2077:i16, "derivative gain (Kc*Td/Ts)"=w2076:i16)
        n1455 = Compound Arithmetic op=AND(w2080, w2091, w2083) -> (w2084:bool)
        n1456 = xnode "Read/Write Control"("FPGA VI Reference In"=w2094, "error in"=w2093, "Red FB Setpoint"=w2085, "Red FB On/Off"=w2084, "RI Current Out"=w2088, "P4"=w2078, "I4"=w2077, "D4"=w2076) -> ("error out"=w2092:errorcluster)  [unwired: 1 out]
      }
      event "+ phase (APD 1 Gate)", "- phase (APD 1 Gate)", "+ phase (APD 2 Gate)", "- phase (APD 2 Gate)", "+ phase (APD 3 Gate)", "- phase (APD 3 Gate)", "+ phase (APD Acq)", "- phase (APD Acq)": Value Change {
        n1457 = event-data() -> ()  [unwired: 7 out]
        n1458 = local read "Phase Adj. (APD 1 Gate)"() -> (w2114:i16)
        n1459 = Or(x="- phase (APD 1 Gate)", y="+ phase (APD 1 Gate)") -> (x .or. y?=w2116:bool)
        n1460 = Negate(x=w2114) -> (-x=w2121:i16)
        n1461 = Select(t=w2121, s="+ phase (APD 1 Gate)", f=w2114) -> (s? t:f=w2120:i16)
        n1462 = local read "Phase Adj. (APD 2 Gate)"() -> (w2111:i16)
        n1463 = Or(x="- phase (APD 2 Gate)", y="+ phase (APD 2 Gate)") -> (x .or. y?=w2109:bool)
        n1464 = Negate(x=w2111) -> (-x=w2113:i16)
        n1465 = Select(t=w2113, s="+ phase (APD 2 Gate)", f=w2111) -> (s? t:f=w2110:i16)
        n1466 = Negate(x="Phase Adj. (APD 3 Gate)") -> (-x=w2108:i16)
        n1467 = Or(x="- phase (APD 3 Gate)", y="+ phase (APD 3 Gate)") -> (x .or. y?=w2104:bool)
        n1468 = Select(t=w2108, s="+ phase (APD 3 Gate)", f="Phase Adj. (APD 3 Gate)") -> (s? t:f=w2105:i16)
        n1469 = local read "Phase Adj. (APD Acq)"() -> (w2102:i16)
        n1470 = Or(x="- phase (APD Acq)", y="+ phase (APD Acq)") -> (x .or. y?=w2100:bool)
        n1471 = Negate(x=w2102) -> (-x=w2103:i16)
        n1472 = Select(t=w2103, s="+ phase (APD Acq)", f=w2102) -> (s? t:f=w2101:i16)
        n1473 = xnode "Read/Write Control"("FPGA VI Reference In"=w2123, "error in"=w2122, "Phase count adjustment (APD 1 Gate)"=w2120, "Phase count adjustment (APD 2 Gate)"=w2110, "Phase count adjustment (APD 3 Gate)"=w2105, "Phase Count Adjustment (APD Acq)"=w2101) -> ("FPGA VI Reference Out"=w2118:T20, "error out"=w2119:errorcluster)
        n1474 = xnode "Read/Write Control"("FPGA VI Reference In"=w2118, "error in"=w2119, "+ phase (APD 1 Gate)"=w2116, "+ phase (APD 2 Gate)"=w2109, "+ phase (APD 3 Gate)"=w2104, "+ phase (APD Acq)"=w2100) -> ("error out"=w2117:errorcluster)  [unwired: 1 out]
      }
      event "Invert APD Gate", "APD Gate ON Count", "APD Gate OFF Count", "APD Gate", "APD Integration Time (s)", "APD AO Scale Factor", "Duty Frequency (ON 1/N cycles)", "Interlace ON count", "Interlace OFF count": Value Change {
        n1475 = event-data() -> ()  [unwired: 7 out]
        n1476 = Add(x="Interlace ON count", y="Interlace OFF count") -> (x+y=w2129:u16)
        n1477 = Add(x="APD Gate ON Count", y="APD Gate OFF Count") -> (x+y=w2140:u16)
        n1478 = Multiply(x="Duty Frequency (ON 1/N cycles)", y=w2129) -> (x*y=w2125:u16)
        "Green AI Count" <- w2125
        "Red AI Count" <- w2125
        "Blue AI Count" <- w2125
        n1479 = Subtract(x=w2125, y="Interlace ON count") -> (x-y=w2128:u16)
        n1480 = Multiply(x=w2140, y="Duty Frequency (ON 1/N cycles)") -> (x*y=w2139:u16)
        n1481 = Subtract(x=w2139, y="APD Gate ON Count") -> (x-y=w2138:u16)
        n1482 = local read "DMA Update Period (s)"() -> (w2141:dbl)
        n1483 = Multiply(x="APD Integration Time (s)", y=40000000.0) -> (x*y=w2145:dbl)
        n1484 = Reciprocal(x="APD Integration Time (s)") -> (1/x=→"APD Acq Rate (Hz)":dbl)
        n1485 = To Unsigned Long Integer(number=w2145) -> (unsigned 32bit integer=w2131:u32)
        "APD Int. Count" <- w2131
        n1486 = local read "Number of APDs"() -> (w2124:u8)
        n1487 = Divide(x=w2141, y="APD Integration Time (s)") -> (x/y=w2143:dbl)
        n1488 = Multiply(x=w2124, y=w2143) -> (x*y=w2142:dbl)
        n1489 = local write "APD Samples/FIFO Acq."(w2143) -> ()
        n1490 = local write "APD Elements/DMA read"(w2142) -> ()
        n1491 = xnode "Read/Write Control"("FPGA VI Reference In"=w2149, "error in"=w2148, "Invert APD Gate"="Invert APD Gate", "APD Gate ON Count"="APD Gate ON Count", "APD Gate OFF Count"=w2138, "APD Acq Rate Count"=w2131, "APD Gate Operating Mode"="APD Gate", "APD AO scale factor"="APD AO Scale Factor", "Green interlace ON count"="Interlace ON count", "Green interlace OFF count"=w2128, "Green interlace ON count 2"="Interlace ON count", "Green interlace OFF count 2"=w2128, "Green FB Count"=w2125, "Red interlace ON count"="Interlace ON count", "Red interlace OFF count"="Interlace OFF count", "Blue ON count (AO)"="Interlace ON count", "Blue OFF count (AO)"="Interlace OFF count", "Blue interlace OFF count (D)"="Interlace OFF count", "Blue interlace ON count (D)"="Interlace ON count") -> ("error out"=w2147:errorcluster)  [unwired: 1 out]
      }
      event "Neg. TTrig FPGA": Value Change {
        n1492 = event-data() -> ()  [unwired: 7 out]
        n1493 = xnode "Read/Write Control"("FPGA VI Reference In"=w2152, "error in"=w2151, "TTrig Negate Pos"="Neg. TTrig FPGA") -> ()  [unwired: 2 out]
      }
      event "Test ttrig": Value Change {
        n1494 = event-data() -> ()  [unwired: 7 out]
        n1495 = xnode "Read/Write Control"("FPGA VI Reference In"=w2156, "error in"=w2155, "TTrig?"=TRUE) -> ("error out"=w2154:errorcluster)  [unwired: 1 out]
      }
      event "Number of F/B Scans (AOD)", "Scan Speed (nm/s)", "Scan BD", "Initial delta (MHz)", "Step Size (nm)", "Scan Range (nm)": Value Change {
        w2219 = 123.0  # AOM cal (nm/MHz)
        n1496 = event-data() -> ()  [unwired: 7 out]
        n1497 = local read "BD 1 Frequency 1 (MHz)"() -> (w2202:dbl)
        n1498 = local read "AOM X Cal (nm/MHz)"() -> (w2194:dbl)
        n1499 = local read "X RF Frequency Limits (MHz)"() -> (w2206:T16)
        n1500 = local read "Y RF Frequency Limits (MHz)"() -> (w2203:T16)
        n1501 = local read "BD 2 Frequency 1 (MHz)"() -> (w2208:dbl)
        n1502 = Negate(x="Scan Range (nm)") -> (-x=w2172:dbl)
        n1503 = Divide(x=w2172, y=w2194) -> (x/y=w2176:dbl)
        n1504 = Select(t=w2206, s="Scan BD", f=w2203) -> (s? t:f=w2205:T16)
        n1505 = Select(t=w2202, s="Scan BD", f=w2208) -> (s? t:f=w2207:dbl)
        n1506 = Unbundle By Name(w2205) -> ("Maximum"=w2214:dbl, "Minimum"=w2213:dbl)
        n1507 = Add(x=w2176, y=w2207) -> (x+y=w2211:dbl)
        n1508 = Divide(x=w2172, y="Step Size (nm)") -> (x/y=w2191:dbl)
        n1509 = Divide(x="Step Size (nm)", y=w2194) -> (x/y=w2200:dbl)
        n1510 = Absolute Value(x=w2191) -> (abs(x)=w2175:dbl)
        n1511 = Sign(1:w2172) -> (0:w2173:dbl)
        n1512 = In Range and Coerce(upper limit=w2214, x=w2211, lower limit=w2213) -> (coerced(x)=w2210:dbl, In Range?=w2212:bool)
        n1513 = To Unsigned Quad Integer(1:w2175) -> (0:w2190:u64)
        "Scan steps (AOD)" <- w2190
        n1514 = call "IR AOM freq to word.vi"("Frequency In (MHz)"=w2200) -> ("Frequency Word Out (double)"=w2197:dbl)
        n1515 = Multiply(x=w2173, y=w2197) -> (x*y=w2174:dbl)
        n1516 = Subtract(x=w2211, y=w2210) -> (x-y=w2209:dbl)
        n1517 = To Quad Integer(1:w2174) -> (0:w2196:i64)
        "Incr. int (AOD)" <- w2196
        n1518 = Subtract(x=w2176, y=w2209) -> (x-y=w2195:dbl)
        "Scan Range (MHz)" <- w2195
        n1519 = Select(t=w2176, s=w2212, f=w2195) -> (s? t:f=w2215:dbl)
        n1520 = Multiply(x=w2195, y=w2194) -> (x*y=w2193:dbl)
        n1521 = Decrement(x=w2190) -> (x-1=w2243:u64)
        n1522 = Negate(x=w2193) -> (-x=w2189:dbl)
        n1523 = local write "Scan Range (nm)"(w2189) -> ()
        n1524 = Divide(x=w2215, y=w2243) -> (x/y=w2199:dbl)
        "Scan Increment (MHz)" <- w2199
        n1525 = call "IR AOM freq to word.vi"("Frequency In (MHz)"=w2199) -> ("Frequency Word Out (double)"=w2198:dbl)
        n1526 = Divide(x="Step Size (nm)", y="Scan Speed (nm/s)") -> (x/y=w2186:dbl)
        n1527 = To Quad Integer(1:w2198) -> ()  [unwired: 1 out]
        n1528 = local read "Number Interlace Sets"() -> (w2170:u8)
        n1529 = local read "AI Count (ticks)"() -> (w2171:u16)
        n1530 = local read "Total Counts (ticks)"() -> (w2169:u16)
        n1531 = local read "# Samples/trap"() -> (w2201:u32)
        n1532 = Multiply(x=w2171, y=w2170) -> (x*y=w2168:u16)
        n1533 = Divide(x=w2169, y=w2168) -> (x/y=w2167:dbl)
        n1534 = Select(t=w2202, s="Scan BD", f=w2208) -> (s? t:f=w2240:dbl)
        "Initial freq. (MHz)" <- w2240
        n1535 = Add(x=w2215, y=w2240) -> (x+y=→"Final freq. (MHz)":dbl)
        n1536 = Divide(x=w2169, y=40000000.0) -> (x/y=w2185:dbl)
        n1537 = Divide(x=w2186, y=w2185) -> (x/y=w2184:dbl)
        n1538 = To Unsigned Quad Integer(1:w2184) -> (0:w2159:u64)
        n1539 = Quotient & Remainder(x=w2159, y=u64 2) -> (x-y*floor(x/y)=w2163:u64)  [unwired: 1 out]
        n1540 = Equal?(x=w2163, y=u64 0) -> (x = y?=w2161:bool)
        n1541 = Decrement(x=w2159) -> (x-1=w2160:u64)
        n1542 = Select(t=w2159, s=w2161, f=w2160) -> (s? t:f=w2158:u64)
        "Cycles/step (AOD)" <- w2158
        n1543 = xnode "Read/Write Control"("FPGA VI Reference In"=w2251, "error in"=w2250, "Scan steps"=w2190, "Number of scans"="Number of F/B Scans (AOD)", "Cycles per step"=w2158, "Scan freq.  increment"=w2196, "Scan BD"="Scan BD") -> ("error out"=w2249:errorcluster)  [unwired: 1 out]
        n1544 = Multiply(x=w2190, y=w2158) -> (x*y=w2244:u64)
        n1545 = Multiply(x=w2244, y=u64 2) -> (x*y=w2166:u64)
        n1546 = Multiply(x=w2167, y=w2166) -> (x*y=w2165:dbl)
        "Data points/scan (f/b)" <- w2165
        n1547 = Multiply(x=w2165, y="Number of F/B Scans (AOD)") -> (x*y=w2247:dbl)
        "Data points/scans" <- w2247
        n1548 = Divide(x=w2247, y=w2201) -> (x/y=→"N sets should be saved":dbl)
        n1549 = Multiply(x=w2244, y=w2185) -> (x*y=w2183:dbl)
        "Time/Scan (s) (AOD)" <- w2183
        n1550 = Select(t=w2215, s="Scan BD", f=0.0) -> (s? t:f=w2241:dbl)
        n1551 = Select(t=0.0, s="Scan BD", f=w2215) -> (s? t:f=w2237:dbl)
        n1552 = local read "BD 2 Frequency 2 (MHz)"() -> (w2233:dbl)
        n1553 = local read "BD 1 Frequency 2 (MHz)"() -> (w2236:dbl)
        n1554 = Add(x=w2237, y=w2208) -> (x+y=w2234:dbl)
        n1555 = Add(x=w2202, y=w2241) -> (x+y=w2235:dbl)
        n1556 = Multiply(x=w2183, y=2.0) -> (x*y=w2182:dbl)